vi "TLB Native Dynamic Events ver 0.26d.vi"() -> ()   [LabVIEW 2018] (continued)
                    n435 = for {
                      tunnel: string[] ["START TIMER", "OPEN CLAW", ""] ("element") -> [w1149] mode=indexing
                      shift-right: [w1151] -> w1148
                      shift-left: w1146 -> [w1150]
                      n436 = Enqueue Element(queue=w1150, element=w1149) -> (queue out=w1151:refnum<queue>)  [unwired: 2 in, 2 out]
                    }
                  }
                  frame True {
                    n437 = for {
                      shift-right: [w1156] -> w1154
                      shift-left: w1152 -> [w1157]
                      tunnel: string[] ["CAM CLOSE", "", ""] -> [w1155] mode=indexing
                      n438 = Enqueue Element(queue=w1157, element=w1155) -> (queue out=w1156:refnum<queue>)  [unwired: 2 in, 2 out]
                    }
                  }
                }
                n439 = Or(x=w1135, y=w1140) -> (x .or. y?=w1142:bool)
                n440 = Select(t=State_Type_Definitions,_for_0.26g_versions_and_later_2."True Stop" ("Enum"), s=w1140, f=State_Type_Definitions,_for_0.26g_versions_and_later_2."True Stop" ("Enum")) -> (s? t:f=w1137:T18)
                n441 = Select(t=w1137, s=w1142, f=State_Type_Definitions,_for_0.26g_versions_and_later_2."Task 5D" ("Enum")) -> (s? t:f=w1141:T18)
              }
              frame "Exit" {
                n442 = for {
                  shift-right: [w1164] -> w1161
                  shift-left: w1158 -> [w1165]
                  tunnel: string[] ["STOP", "RESET ENCODERS", "RESET YAW", "ARDUINO MODE 0"] -> [w1163] mode=indexing
                  n443 = Enqueue Element(queue=w1165, element=w1163) -> (queue out=w1164:refnum<queue>)  [unwired: 2 in, 2 out]
                }
              }
            }
          }
          frame 20 {
            # ">>> yStepper command>>>"
            n444 = Dequeue Element(queue=w1179, timeout in ms (-1)=w1180, error in (no error)=w1181) -> (element=w1183:T10)  [unwired: 3 out]
            n445 = formula code="if (pos < 100)\ny = 41;\n\nelse if (pos >= 100 && pos <= 140)\ny = 30;\n\nelse if (pos >= 141 && pos <= 170)\ny = 25;\n\nelse if (pos >= 171 &&pos <= 180) \ny = 20;\n\nelse if (pos >= 181&& pos <= 200)\ny = 15;\n\nelse if (pos >= 201 && pos <= 230)\ny = 10;\n\nelse if (pos >= 231 && pos <= 320)\ny = 8;\n\nelse if (pos > 320)\ny = 0;"("pos"=w1171) -> ("y"=w1174:dbl)
            n446 = To Unsigned Byte Integer(number=w1174) -> (unsigned 8bit integer=w1169:u8)
            n447 = Equal?(x=w1170, y=w1169) -> (x = y?=w1168:bool)
            n448 = case shown="\"Start Task 1\", Default" w1183 {
              tunnel: [w1190 State_Type_Definitions,_for_0.26g_versions_and_later_2."True Stop" ("Enum")] -> w1177
              tunnel: [w1193 w1210] -> w1175
              tunnel: [State_Type_Definitions,_for_0.26g_versions_and_later_2."Idle" ("Enum") State_Type_Definitions,_for_0.26g_versions_and_later_2."Shutdown" ("Enum")] -> w1176
              tunnel: w1182 -> [w1189 _]
              tunnel: w1178 -> [w1185 w1207]
              tunnel: w1168 -> [w1184 _]
              frame "Start Task 1", Default {
                # ">> T: Breaks out of state loop; F: Stays in loop>>"
                # ">> Manual override >>"
                # ">> Checks if time is up>>"
                # "Stays in Task 5D until the object is detected"
                # "T: Go back to idle, F: Continue with task\""
                # ">> Manual override >>"
                n449 = case shown="False" w1184 {
                  tunnel: [w1197 w1203] -> w1193
                  tunnel: w1185 -> [w1195 w1201]
                  frame False {
                    n450 = for {
                      tunnel: string[] ["READ STEPPER VALUES", "Y STEPPER CONTROL", ""] ("element") -> [w1198] mode=indexing
                      shift-right: [w1200] -> w1197
                      shift-left: w1195 -> [w1199]
                      n451 = Enqueue Element(queue=w1199, element=w1198) -> (queue out=w1200:refnum<queue>)  [unwired: 2 in, 2 out]
                    }
                  }
                  frame True {
                    n452 = for {
                      shift-right: [w1205] -> w1203
                      shift-left: w1201 -> [w1206]
                      tunnel: string[] ["CAM CLOSE", "DISPOSE BUFFERS", ""] -> [w1204] mode=indexing
                      n453 = Enqueue Element(queue=w1206, element=w1204) -> (queue out=w1205:refnum<queue>)  [unwired: 2 in, 2 out]
                    }
                  }
                }
                n454 = Or(x=w1184, y=w1189) -> (x .or. y?=w1191:bool)
                n455 = Select(t=State_Type_Definitions,_for_0.26g_versions_and_later_2."True Stop" ("Enum"), s=w1189, f=State_Type_Definitions,_for_0.26g_versions_and_later_2."Task 5F: ARM GRAB HEIGHT" ("Enum")) -> (s? t:f=w1186:T18)
                n456 = Select(t=w1186, s=w1191, f=State_Type_Definitions,_for_0.26g_versions_and_later_2."Task 5E: POSITION ARM" ("Enum")) -> (s? t:f=w1190:T18)
              }
              frame "Exit" {
                n457 = for {
                  shift-right: [w1213] -> w1210
                  shift-left: w1207 -> [w1214]
                  tunnel: string[] ["STOP", "RESET ENCODERS", "RESET YAW", "ARDUINO MODE 0"] -> [w1212] mode=indexing
                  n458 = Enqueue Element(queue=w1214, element=w1212) -> (queue out=w1213:refnum<queue>)  [unwired: 2 in, 2 out]
                }
              }
            }
            n459 = Bundle By Name(cluster=w1173, "yStepper desired"=w1169) -> (w1172:T20)
          }
          frame 21 {
            # ">>> Motor control cluster >>>"
            # ">>> yStepper command>>>"
            # ">> Manual override >>"
            n460 = Dequeue Element(queue=w1225, timeout in ms (-1)=w1224, error in (no error)=w1226) -> (element=w1223:T10)  [unwired: 3 out]
            n461 = Equal?(x=w1222, y=u8 1) -> (x = y?=w1220:bool)
            n462 = case shown="\"Start Task 1\", Default" w1223 {
              tunnel: [w1236 State_Type_Definitions,_for_0.26g_versions_and_later_2."True Stop" ("Enum")] -> w1227
              tunnel: [w1239 w1256] -> w1228
              tunnel: [State_Type_Definitions,_for_0.26g_versions_and_later_2."Idle" ("Enum") State_Type_Definitions,_for_0.26g_versions_and_later_2."Shutdown" ("Enum")] -> w1229
              tunnel: w1220 -> [w1235 _]
              tunnel: w1219 -> [w1234 _]
              tunnel: w1218 -> [w1230 w1253]
              frame "Start Task 1", Default {
                # "Stays in Task 5F until stepper reaches desired \nheight"
                # "T: Go back to idle, F: Continue with task\""
                # ">> Manual override >>"
                n463 = case shown="True" w1235 {
                  tunnel: [w1243 w1249] -> w1239
                  tunnel: w1230 -> [w1241 w1247]
                  frame False {
                    n464 = for {
                      tunnel: string[] ["Z STEPPER GRAB HEIGHT", "READ STEPPER VALUES"] ("element") -> [w1244] mode=indexing
                      shift-right: [w1246] -> w1243
                      shift-left: w1241 -> [w1245]
                      n465 = Enqueue Element(queue=w1245, element=w1244) -> (queue out=w1246:refnum<queue>)  [unwired: 2 in, 2 out]
                    }
                  }
                  frame True {
                    n466 = for {
                      shift-right: [w1251] -> w1249
                      shift-left: w1247 -> [w1252]
                      tunnel: string[] ["SET TIMER 5", "CLOSE CLAW", ""] -> [w1250] mode=indexing
                      n467 = Enqueue Element(queue=w1252, element=w1250) -> (queue out=w1251:refnum<queue>)  [unwired: 2 in, 2 out]
                    }
                  }
                }
                n468 = Or(x=w1235, y=w1234) -> (x .or. y?=w1237:bool)
                n469 = Select(t=State_Type_Definitions,_for_0.26g_versions_and_later_2."True Stop" ("Enum"), s=w1234, f=State_Type_Definitions,_for_0.26g_versions_and_later_2."Task 5G: CLOSE CLAW" ("Enum")) -> (s? t:f=w1231:T18)
                n470 = Select(t=w1231, s=w1237, f=State_Type_Definitions,_for_0.26g_versions_and_later_2."Task 5F: ARM GRAB HEIGHT" ("Enum")) -> (s? t:f=w1236:T18)
              }
              frame "Exit" {
                n471 = for {
                  shift-right: [w1259] -> w1256
                  shift-left: w1253 -> [w1260]
                  tunnel: string[] ["STOP", "RESET ENCODERS", "RESET YAW", "ARDUINO MODE 0"] -> [w1258] mode=indexing
                  n472 = Enqueue Element(queue=w1260, element=w1258) -> (queue out=w1259:refnum<queue>)  [unwired: 2 in, 2 out]
                }
              }
            }
          }
          frame 22 {
            # ">>> yStepper command>>>"
            # ">> Manual override >>"
            n473 = Dequeue Element(queue=w1271, timeout in ms (-1)=w1270, error in (no error)=w1269) -> (element=w1268:T10)  [unwired: 3 out]
            n474 = case shown="\"Start Task 1\", Default" w1268 {
              tunnel: [w1280 State_Type_Definitions,_for_0.26g_versions_and_later_2."True Stop" ("Enum")] -> w1273
              tunnel: [w1283 w1300] -> w1266
              tunnel: [State_Type_Definitions,_for_0.26g_versions_and_later_2."Idle" ("Enum") State_Type_Definitions,_for_0.26g_versions_and_later_2."Shutdown" ("Enum")] -> w1265
              tunnel: w1267 -> [w1274 _]
              tunnel: w1272 -> [w1279 w1297]
              tunnel: w1263 -> [w1278 _]
              frame "Start Task 1", Default {
                # ">> Is time up? >>"
                # "Determines if object is in range to pick up"
                # ">> Manual override >>"
                n475 = case shown="True" w1278 {
                  tunnel: [w1287 w1293] -> w1283
                  tunnel: w1279 -> [w1285 w1291]
                  frame False {
                    n476 = for {
                      tunnel: string[] ["CLOSE CLAW", "START TIMER"] ("element") -> [w1288] mode=indexing
                      shift-right: [w1290] -> w1287
                      shift-left: w1285 -> [w1289]
                      n477 = Enqueue Element(queue=w1289, element=w1288) -> (queue out=w1290:refnum<queue>)  [unwired: 2 in, 2 out]
                    }
                  }
                  frame True {
                    n478 = for {
                      shift-right: [w1295] -> w1293
                      shift-left: w1291 -> [w1296]
                      tunnel: string[] ["READ STEPPER VALUES", "", ""] -> [w1294] mode=indexing
                      n479 = Enqueue Element(queue=w1296, element=w1294) -> (queue out=w1295:refnum<queue>)  [unwired: 2 in, 2 out]
                    }
                  }
                }
                n480 = Or(x=w1278, y=w1274) -> (x .or. y?=w1281:bool)
                n481 = Select(t=State_Type_Definitions,_for_0.26g_versions_and_later_2."True Stop" ("Enum"), s=w1274, f=State_Type_Definitions,_for_0.26g_versions_and_later_2."Task 5H: RAISE ARM" ("Enum")) -> (s? t:f=w1276:T18)
                n482 = Select(t=w1276, s=w1281, f=State_Type_Definitions,_for_0.26g_versions_and_later_2."Task 5G: CLOSE CLAW" ("Enum")) -> (s? t:f=w1280:T18)
              }
              frame "Exit" {
                n483 = for {
                  shift-right: [w1303] -> w1300
                  shift-left: w1297 -> [w1304]
                  tunnel: string[] ["STOP", "RESET ENCODERS", "RESET YAW", "ARDUINO MODE 0"] -> [w1302] mode=indexing
                  n484 = Enqueue Element(queue=w1304, element=w1302) -> (queue out=w1303:refnum<queue>)  [unwired: 2 in, 2 out]
                }
              }
            }
          }
          frame 23 {
            # ">>> yStepper command>>>"
            # ">> Manual override >>"
            n485 = Dequeue Element(queue=w1315, timeout in ms (-1)=w1314, error in (no error)=w1316) -> (element=w1313:T10)  [unwired: 3 out]
            n486 = Equal?(x=w1312, y=u8 60) -> (x = y?=w1310:bool)
            n487 = case shown="\"Start Task 1\", Default" w1313 {
              tunnel: [w1326 State_Type_Definitions,_for_0.26g_versions_and_later_2."True Stop" ("Enum")] -> w1317
              tunnel: [w1329 w1346] -> w1318
              tunnel: [State_Type_Definitions,_for_0.26g_versions_and_later_2."Idle" ("Enum") State_Type_Definitions,_for_0.26g_versions_and_later_2."Shutdown" ("Enum")] -> w1319
              tunnel: w1310 -> [w1325 _]
              tunnel: w1309 -> [w1324 _]
              tunnel: w1308 -> [w1320 w1343]
              frame "Start Task 1", Default {
                # "Stays in Task 5_A until stepper reaches desired \nheight"
                # "T: Go back to idle, F: Continue with task\""
                # ">> Manual override >>"
                n488 = case shown="False" w1325 {
                  tunnel: [w1333 w1339] -> w1329
                  tunnel: w1320 -> [w1331 w1337]
                  frame False {
                    n489 = for {
                      tunnel: string[] ["Z STEPPER CAM HEIGHT", "READ STEPPER VALUES"] ("element") -> [w1334] mode=indexing
                      shift-right: [w1336] -> w1333
                      shift-left: w1331 -> [w1335]
                      n490 = Enqueue Element(queue=w1335, element=w1334) -> (queue out=w1336:refnum<queue>)  [unwired: 2 in, 2 out]
                    }
                  }
                  frame True {
                    n491 = for {
                      shift-right: [w1341] -> w1339
                      shift-left: w1337 -> [w1342]
                      tunnel: string[] ["ARDUINO - ULTRASONIC", "READ ULTRASONIC", ""] -> [w1340] mode=indexing
                      n492 = Enqueue Element(queue=w1342, element=w1340) -> (queue out=w1341:refnum<queue>)  [unwired: 2 in, 2 out]
                    }
                  }
                }
                n493 = Or(x=w1325, y=w1324) -> (x .or. y?=w1327:bool)
                n494 = Select(t=State_Type_Definitions,_for_0.26g_versions_and_later_2."True Stop" ("Enum"), s=w1324, f=State_Type_Definitions,_for_0.26g_versions_and_later_2."True Stop" ("Enum")) -> (s? t:f=w1321:T18)
                n495 = Select(t=w1321, s=w1327, f=State_Type_Definitions,_for_0.26g_versions_and_later_2."Task 5H: RAISE ARM" ("Enum")) -> (s? t:f=w1326:T18)
              }
              frame "Exit" {
                n496 = for {
                  shift-right: [w1349] -> w1346
                  shift-left: w1343 -> [w1350]
                  tunnel: string[] ["STOP", "RESET ENCODERS", "RESET YAW", "ARDUINO MODE 0"] -> [w1348] mode=indexing
                  n497 = Enqueue Element(queue=w1350, element=w1348) -> (queue out=w1349:refnum<queue>)  [unwired: 2 in, 2 out]
                }
              }
            }
          }
          frame 24 {
            # ">>> yStepper command>>>"
            n498 = Dequeue Element(queue=w1360, timeout in ms (-1)=w1359, error in (no error)=w1358) -> (element=w1365:T10)  [unwired: 3 out]
            n499 = Equal?(x=w1356, y=u8 60) -> (x = y?=w1355:bool)
            n500 = case shown="\"Start Task 1\", Default" w1365 {
              tunnel: [w1372 State_Type_Definitions,_for_0.26g_versions_and_later_2."True Stop" ("Enum")] -> w1363
              tunnel: [w1371 w1389] -> w1362
              tunnel: [State_Type_Definitions,_for_0.26g_versions_and_later_2."Idle" ("Enum") State_Type_Definitions,_for_0.26g_versions_and_later_2."Shutdown" ("Enum")] -> w1364
              tunnel: w1361 -> [w1367 _]
              tunnel: w1357 -> [w1369 _]
              tunnel: w1355 -> [w1366 _]
              frame "Start Task 1", Default {
                n501 = case shown="False" w1366 {
                  tunnel: [w1377 w1383] -> w1371
                  tunnel: w1369 -> [w1375 w1381]
                  frame False {
                    n502 = for {
                      tunnel: string[] ["Z STEPPER CAM HEIGHT", "READ STEPPER VALUES"] ("element") -> [w1378] mode=indexing
                      shift-right: [w1380] -> w1377
                      shift-left: w1375 -> [w1379]
                      n503 = Enqueue Element(queue=w1379, element=w1378) -> (queue out=w1380:refnum<queue>)  [unwired: 2 in, 2 out]
                    }
                  }
                  frame True {
                    n504 = for {
                      shift-right: [w1385] -> w1383
                      shift-left: w1381 -> [w1386]
                      tunnel: string[] ["CAM ACQ", "OPEN LOG CAM"] -> [w1384] mode=indexing
                      n505 = Enqueue Element(queue=w1386, element=w1384) -> (queue out=w1385:refnum<queue>)  [unwired: 2 in, 2 out]
                    }
                  }
                }
                n506 = Or(x=w1366, y=w1367) -> (x .or. y?=w1368:bool)
                n507 = Select(t=State_Type_Definitions,_for_0.26g_versions_and_later_2."Task 6_B" ("Enum"), s=w1368, f=State_Type_Definitions,_for_0.26g_versions_and_later_2."Task 6_A" ("Enum")) -> (s? t:f=w1372:T18)
              }
              frame "Exit" {
                n508 = for {
                  shift-right: [w1392] -> w1389
                  shift-left: _ -> [w1393]
                  tunnel: string[] ["STOP", "RESET ENCODERS", "RESET YAW", "ARDUINO MODE 0"] -> [w1391] mode=indexing
                  n509 = Enqueue Element(queue=w1393, element=w1391) -> (queue out=w1392:refnum<queue>)  [unwired: 2 in, 2 out]
                }
              }
            }
          }
          frame 25 {
            # ">>> yStepper command>>>"
            n510 = Dequeue Element(queue=w1405, timeout in ms (-1)=w1403, error in (no error)=w1404) -> (element=w1402:T10)  [unwired: 3 out]
            n511 = case shown="\"Start Task 1\", Default" w1402 {
              tunnel: [w1412 State_Type_Definitions,_for_0.26g_versions_and_later_2."True Stop" ("Enum")] -> w1398
              tunnel: [w1411 w1430] -> w1406
              tunnel: [State_Type_Definitions,_for_0.26g_versions_and_later_2."Idle" ("Enum") State_Type_Definitions,_for_0.26g_versions_and_later_2."Shutdown" ("Enum")] -> w1399
              tunnel: w1401 -> [w1407 _]
              tunnel: w1400 -> [w1409 _]
              tunnel: w1397 -> [w1408 w1427]
              frame "Start Task 1", Default {
                # ">> Manual override >>"
                n512 = case shown="False" w1409 {
                  tunnel: [w1417 w1423] -> w1411
                  tunnel: w1408 -> [w1416 w1421]
                  frame False {
                    n513 = for {
                      shift-right: [w1420] -> w1417
                      shift-left: w1416 -> [w1419]
                      tunnel: string[] ["CAM ACQ", "PROCESS IMAGE", "OPEN CLAW"] -> [w1418] mode=indexing
                      n514 = Enqueue Element(queue=w1419, element=w1418) -> (queue out=w1420:refnum<queue>)  [unwired: 2 in, 2 out]
                    }
                  }
                  frame True {
                    n515 = for {
                      shift-right: [w1425] -> w1423
                      shift-left: w1421 -> [w1426]
                      tunnel: string[] ["CAM ACQ", "PROCESS IMAGE", "CLOSE CLAW"] -> [w1424] mode=indexing
                      n516 = Enqueue Element(queue=w1426, element=w1424) -> (queue out=w1425:refnum<queue>)  [unwired: 2 in, 2 out]
                    }
                  }
                }
                n517 = Select(t=State_Type_Definitions,_for_0.26g_versions_and_later_2."True Stop" ("Enum"), s=w1407, f=State_Type_Definitions,_for_0.26g_versions_and_later_2."Task 6_B" ("Enum")) -> (s? t:f=w1412:T18)
              }
              frame "Exit" {
                # ">> State after true stop >>"
                # ">> Goes to true stop >>"
                n518 = for {
                  shift-right: [w1433] -> w1430
                  shift-left: w1427 -> [w1434]
                  tunnel: string[] ["STOP", "RESET ENCODERS", "RESET YAW", ""] -> [w1432] mode=indexing
                  n519 = Enqueue Element(queue=w1434, element=w1432) -> (queue out=w1433:refnum<queue>)  [unwired: 2 in, 2 out]
                }
              }
            }
          }
          frame 26 {
          }
          frame 27 {
            # ">>> Motor control cluster >>>"
            # ">>> yStepper command>>>"
            # ">> Manual override >>"
            n520 = Dequeue Element(queue=w1451, timeout in ms (-1)=w1450, error in (no error)=w1452) -> (element=w1449:T10)  [unwired: 3 out]
            n521 = Equal?(x=w1448, y=u8 60) -> (x = y?=w1446:bool)
            n522 = case shown="\"Start Task 1\", Default" w1449 {
              tunnel: [w1462 State_Type_Definitions,_for_0.26g_versions_and_later_2."True Stop" ("Enum")] -> w1453
              tunnel: [w1465 w1482] -> w1454
              tunnel: [State_Type_Definitions,_for_0.26g_versions_and_later_2."Idle" ("Enum") State_Type_Definitions,_for_0.26g_versions_and_later_2."Shutdown" ("Enum")] -> w1455
              tunnel: w1446 -> [w1461 _]
              tunnel: w1445 -> [w1460 _]
              tunnel: w1444 -> [w1456 w1479]
              frame "Start Task 1", Default {
                # "Stays in Task 5_A until stepper reaches desired \nheight"
                # "T: Go back to idle, F: Continue with task\""
                # ">> Manual override >>"
                n523 = case shown="False" w1461 {
                  tunnel: [w1469 w1475] -> w1465
                  tunnel: w1456 -> [w1467 w1473]
                  frame False {
                    n524 = for {
                      tunnel: string[] ["Z STEPPER CAM HEIGHT", "READ STEPPER VALUES"] ("element") -> [w1470] mode=indexing
                      shift-right: [w1472] -> w1469
                      shift-left: w1467 -> [w1471]
                      n525 = Enqueue Element(queue=w1471, element=w1470) -> (queue out=w1472:refnum<queue>)  [unwired: 2 in, 2 out]
                    }
                  }
                  frame True {
                    n526 = for {
                      shift-right: [w1477] -> w1475
                      shift-left: w1473 -> [w1478]
                      tunnel: string[] ["ARDUINO - ULTRASONIC", "READ ULTRASONIC", ""] -> [w1476] mode=indexing
                      n527 = Enqueue Element(queue=w1478, element=w1476) -> (queue out=w1477:refnum<queue>)  [unwired: 2 in, 2 out]
                    }
                  }
                }
                n528 = Or(x=w1461, y=w1460) -> (x .or. y?=w1463:bool)
                n529 = Select(t=State_Type_Definitions,_for_0.26g_versions_and_later_2."True Stop" ("Enum"), s=w1460, f=State_Type_Definitions,_for_0.26g_versions_and_later_2."Task 8B: MOVE TO BOX" ("Enum")) -> (s? t:f=w1457:T18)
                n530 = Select(t=w1457, s=w1463, f=State_Type_Definitions,_for_0.26g_versions_and_later_2."Task 8A: RAISE ARM" ("Enum")) -> (s? t:f=w1462:T18)
              }
              frame "Exit" {
                n531 = for {
                  shift-right: [w1485] -> w1482
                  shift-left: w1479 -> [w1486]
                  tunnel: string[] ["STOP", "RESET ENCODERS", "RESET YAW", "ARDUINO MODE 0"] -> [w1484] mode=indexing
                  n532 = Enqueue Element(queue=w1486, element=w1484) -> (queue out=w1485:refnum<queue>)  [unwired: 2 in, 2 out]
                }
              }
            }
          }
          frame 28 {
            w1494 = u8 15 ("y")
            # ">>> yStepper command>>>"
            n533 = Less?(x=w1491, y=w1494) -> (x < y?=w1492:bool)
            n534 = Dequeue Element(queue=w1498, timeout in ms (-1)=w1497, error in (no error)=w1499) -> (element=w1496:T10)  [unwired: 3 out]
            n535 = Less?(x=w1490, y=w1494) -> (x < y?=w1493:bool)
            n536 = And(x=w1493, y=w1492) -> (x .and. y?=w1489:bool)
            n537 = case shown="\"Start Task 1\", Default" w1496 {
              tunnel: [w1511 State_Type_Definitions,_for_0.26g_versions_and_later_2."True Stop" ("Enum")] -> w1501
              tunnel: [w1514 w1531] -> w1500
              tunnel: [State_Type_Definitions,_for_0.26g_versions_and_later_2."Idle" ("Enum") State_Type_Definitions,_for_0.26g_versions_and_later_2."Shutdown" ("Enum")] -> w1502
              tunnel: w1504 -> [w1510 _]
              tunnel: w1503 -> [w1506 w1528]
              tunnel: w1489 -> [w1505 _]
              frame "Start Task 1", Default {
                # "Stays in Task 5_B to capture image over 5 seconds"
                # "T: Go back to idle, F: Continue with task\""
                # ">> Manual override >>"
                n538 = case shown="True" w1505 {
                  tunnel: [w1518 w1524] -> w1514
                  tunnel: w1506 -> [w1516 w1522]
                  frame False {
                    n539 = for {
                      tunnel: string[] ["FORWARD", "READ ULTRASONIC", "READ NAVX"] ("element") -> [w1519] mode=indexing
                      shift-right: [w1521] -> w1518
                      shift-left: w1516 -> [w1520]
                      n540 = Enqueue Element(queue=w1520, element=w1519) -> (queue out=w1521:refnum<queue>)  [unwired: 2 in, 2 out]
                    }
                  }
                  frame True {
                    n541 = for {
                      shift-right: [w1526] -> w1524
                      shift-left: w1522 -> [w1527]
                      tunnel: string[] ["STOP", "RESET ENCODERS", "OPEN LOG CAM", "SET TIMER 2", "OPEN IMAQ REF"] -> [w1525] mode=indexing
                      n542 = Enqueue Element(queue=w1527, element=w1525) -> (queue out=w1526:refnum<queue>)  [unwired: 2 in, 2 out]
                    }
                  }
                }
                n543 = Or(x=w1505, y=w1510) -> (x .or. y?=w1512:bool)
                n544 = Select(t=State_Type_Definitions,_for_0.26g_versions_and_later_2."True Stop" ("Enum"), s=w1510, f=State_Type_Definitions,_for_0.26g_versions_and_later_2."Task 8C: CAM BURST" ("Enum")) -> (s? t:f=w1507:T18)
                n545 = Select(t=w1507, s=w1512, f=State_Type_Definitions,_for_0.26g_versions_and_later_2."Task 8B: MOVE TO BOX" ("Enum")) -> (s? t:f=w1511:T18)
              }
              frame "Exit" {
                n546 = for {
                  shift-right: [w1534] -> w1531
                  shift-left: w1528 -> [w1535]
                  tunnel: string[] ["STOP", "RESET ENCODERS", "RESET YAW", "ARDUINO MODE 0"] -> [w1533] mode=indexing
                  n547 = Enqueue Element(queue=w1535, element=w1533) -> (queue out=w1534:refnum<queue>)  [unwired: 2 in, 2 out]
                }
              }
            }
          }
          frame 29 {
            # ">>> Motor control cluster >>>"
            # ">>> yStepper command>>>"
            # ">> Manual override >>"
            n548 = Dequeue Element(queue=w1546, timeout in ms (-1)=w1545, error in (no error)=w1544) -> (element=w1543:T10)  [unwired: 3 out]
            n549 = case shown="\"Start Task 1\", Default" w1543 {
              tunnel: [w1555 State_Type_Definitions,_for_0.26g_versions_and_later_2."True Stop" ("Enum")] -> w1548
              tunnel: [w1558 w1575] -> w1541
              tunnel: [State_Type_Definitions,_for_0.26g_versions_and_later_2."Idle" ("Enum") State_Type_Definitions,_for_0.26g_versions_and_later_2."Shutdown" ("Enum")] -> w1540
              tunnel: w1542 -> [w1549 _]
              tunnel: w1547 -> [w1554 w1572]
              tunnel: w1538 -> [w1553 _]
              frame "Start Task 1", Default {
                # ">> Is time up? >>"
                # "Determines if object is in range to pick up"
                # ">> Manual override >>"
                n550 = case shown="True" w1553 {
                  tunnel: [w1562 w1568] -> w1558
                  tunnel: w1554 -> [w1560 w1566]
                  frame False {
                    n551 = for {
                      tunnel: string[] ["CAM ACQ", "START TIMER"] ("element") -> [w1563] mode=indexing
                      shift-right: [w1565] -> w1562
                      shift-left: w1560 -> [w1564]
                      n552 = Enqueue Element(queue=w1564, element=w1563) -> (queue out=w1565:refnum<queue>)  [unwired: 2 in, 2 out]
                    }
                  }
                  frame True {
                    n553 = for {
                      shift-right: [w1570] -> w1568
                      shift-left: w1566 -> [w1571]
                      tunnel: string[] ["CAM CLOSE", "PROCESS IMAGE", "SET TIMER 5"] -> [w1569] mode=indexing
                      n554 = Enqueue Element(queue=w1571, element=w1569) -> (queue out=w1570:refnum<queue>)  [unwired: 2 in, 2 out]
                    }
                  }
                }
                n555 = Or(x=w1553, y=w1549) -> (x .or. y?=w1556:bool)
                n556 = Select(t=State_Type_Definitions,_for_0.26g_versions_and_later_2."True Stop" ("Enum"), s=w1549, f=State_Type_Definitions,_for_0.26g_versions_and_later_2."Task 8D: PROCESS IMAGE" ("Enum")) -> (s? t:f=w1551:T18)
                n557 = Select(t=w1551, s=w1556, f=State_Type_Definitions,_for_0.26g_versions_and_later_2."Task 8C: CAM BURST" ("Enum")) -> (s? t:f=w1555:T18)
              }
              frame "Exit" {
                n558 = for {
                  shift-right: [w1578] -> w1575
                  shift-left: w1572 -> [w1579]
                  tunnel: string[] ["STOP", "RESET ENCODERS", "RESET YAW", "ARDUINO MODE 0"] -> [w1577] mode=indexing
                  n559 = Enqueue Element(queue=w1579, element=w1577) -> (queue out=w1578:refnum<queue>)  [unwired: 2 in, 2 out]
                }
              }
            }
          }
          frame 30 {
            # ">>> yStepper command>>>"
            n560 = Dequeue Element(queue=w1587, timeout in ms (-1)=w1586, error in (no error)=w1585) -> (element=w1584:T10)  [unwired: 3 out]
            n561 = case shown="\"Start Task 1\", Default" w1584 {
              tunnel: [w1599 State_Type_Definitions,_for_0.26g_versions_and_later_2."True Stop" ("Enum")] -> w1591
              tunnel: [w1602 w1619] -> w1590
              tunnel: [State_Type_Definitions,_for_0.26g_versions_and_later_2."Idle" ("Enum") State_Type_Definitions,_for_0.26g_versions_and_later_2."Shutdown" ("Enum")] -> w1592
              tunnel: w1588 -> [w1598 _]
              tunnel: w1589 -> [w1594 w1616]
              tunnel: w1582 -> [w1593 _]
              frame "Start Task 1", Default {
                # ">> T: Breaks out of state loop; F: Stays in loop>>"
                # ">> Manual override >>"
                # ">> Checks if time is up>>"
                # "Stays in Task 5D until the object is detected"
                # "T: Go back to idle, F: Continue with task\""
                # ">> Manual override >>"
                n562 = case shown="False" w1593 {
                  tunnel: [w1606 w1612] -> w1602
                  tunnel: w1594 -> [w1604 w1610]
                  frame False {
                    n563 = for {
                      tunnel: string[] ["START TIMER", "PROCESS IMAGE", ""] ("element") -> [w1607] mode=indexing
                      shift-right: [w1609] -> w1606
                      shift-left: w1604 -> [w1608]
                      n564 = Enqueue Element(queue=w1608, element=w1607) -> (queue out=w1609:refnum<queue>)  [unwired: 2 in, 2 out]
                    }
                  }
                  frame True {
                    n565 = for {
                      shift-right: [w1614] -> w1612
                      shift-left: w1610 -> [w1615]
                      tunnel: string[] ["RESET ENCODERS", "", ""] -> [w1613] mode=indexing
                      n566 = Enqueue Element(queue=w1615, element=w1613) -> (queue out=w1614:refnum<queue>)  [unwired: 2 in, 2 out]
                    }
                  }
                }
                n567 = Or(x=w1593, y=w1598) -> (x .or. y?=w1600:bool)
                n568 = Select(t=State_Type_Definitions,_for_0.26g_versions_and_later_2."True Stop" ("Enum"), s=w1598, f=State_Type_Definitions,_for_0.26g_versions_and_later_2."Task 8E: ROBOT ADJUST" ("Enum")) -> (s? t:f=w1595:T18)
                n569 = Select(t=w1595, s=w1600, f=State_Type_Definitions,_for_0.26g_versions_and_later_2."Task 8D: PROCESS IMAGE" ("Enum")) -> (s? t:f=w1599:T18)
              }
              frame "Exit" {
                n570 = for {
                  shift-right: [w1622] -> w1619
                  shift-left: w1616 -> [w1623]
                  tunnel: string[] ["STOP", "RESET ENCODERS", "RESET YAW", "ARDUINO MODE 0"] -> [w1621] mode=indexing
                  n571 = Enqueue Element(queue=w1623, element=w1621) -> (queue out=w1622:refnum<queue>)  [unwired: 2 in, 2 out]
                }
              }
            }
          }
          frame 31 {
            # ">>> Motor control cluster >>>"
            # ">>> yStepper command>>>"
            n572 = Dequeue Element(queue=w1640, timeout in ms (-1)=w1639, error in (no error)=w1638) -> (element=w1637:T10)  [unwired: 3 out]
            n573 = Subtract(x=w1635, y=300.0) -> (x-y=w1633:dbl)
            n574 = formula code="if (error <= -61&&error > -300){\ndistance = -15;\nxSpeed = -30;\n}\n\nelse if (error <= -51 && error >= -60){\ndistance = -10;\nxSpeed = -30;\n}\n\nelse if (error >= -50 && error <= 50){\ndistance = 0;\nxSpeed = 0;\n}\n\nelse if (error >= 51 && error <= 80){\ndistance = 10;\nxSpeed = 30;\n}\n\nelse if (error >= 81 && error <= 100){\ndistance = 15;\nxSpeed = 30;\n}\n\nelse if (error >= 101 && error <= 120){\ndistance = 20;\nxSpeed = 30;\n}\n\nelse if (error >= 121 && error < 300){\ndistance = 25;\nxSpeed = 30;\n}\n\nelse{\ndistance = 0;\nxSpeed = 0;\n}"("error"=w1633) -> ("distance"=w1628:dbl, "xSpeed"=w1630:dbl)
            n575 = formula code="if (target > 0){\nif (current  >= target)\noutput = 1;\n\nelse if (current != target)\noutput = 0;\n}\n\nelse if (target == 0){\nif (current == target)\noutput = 1;\n\nelse if (current != target)\noutput = 0;\n}\n\nelse if (target < 0){\nif (current <= target)\noutput = 1;\n\nelse if (current != target)\noutput = 0;\n}\n\nelse if (current != target)\noutput = 0;"("target"=w1628, "current"=w1629) -> ("output"=w1627:dbl)
            n576 = Bundle By Name(cluster=w1632, "xSpeed"=w1630) -> (w1631:T19)
            n577 = Equal?(x=w1627, y=1.0) -> (x = y?=w1625:bool)
            n578 = case shown="\"Start Task 1\", Default" w1637 {
              tunnel: [w1652 State_Type_Definitions,_for_0.26g_versions_and_later_2."True Stop" ("Enum")] -> w1644
              tunnel: [w1655 w1672] -> w1643
              tunnel: [State_Type_Definitions,_for_0.26g_versions_and_later_2."Idle" ("Enum") State_Type_Definitions,_for_0.26g_versions_and_later_2."Shutdown" ("Enum")] -> w1645
              tunnel: w1641 -> [w1651 _]
              tunnel: w1642 -> [w1647 w1669]
              tunnel: w1625 -> [w1646 _]
              frame "Start Task 1", Default {
                # ">> T: Breaks out of state loop; F: Stays in loop>>"
                # ">> Manual override >>"
                # ">> Checks if time is up>>"
                # "Stays in Task 5D until the object is detected"
                # "T: Go back to idle, F: Continue with task\""
                # ">> Manual override >>"
                n579 = case shown="True" w1646 {
                  tunnel: [w1659 w1665] -> w1655
                  tunnel: w1647 -> [w1657 w1663]
                  frame False {
                    n580 = for {
                      tunnel: string[] ["X AXIS - SLOW", "READ ENCODERS", "READ NAVX"] ("element") -> [w1660] mode=indexing
                      shift-right: [w1662] -> w1659
                      shift-left: w1657 -> [w1661]
                      n581 = Enqueue Element(queue=w1661, element=w1660) -> (queue out=w1662:refnum<queue>)  [unwired: 2 in, 2 out]
                    }
                  }
                  frame True {
                    n582 = for {
                      shift-right: [w1667] -> w1665
                      shift-left: w1663 -> [w1668]
                      tunnel: string[] ["SET TIMER 2", "STOP", "READ STEPPER VALUES", ""] -> [w1666] mode=indexing
                      n583 = Enqueue Element(queue=w1668, element=w1666) -> (queue out=w1667:refnum<queue>)  [unwired: 2 in, 2 out]
                    }
                  }
                }
                n584 = Or(x=w1646, y=w1651) -> (x .or. y?=w1653:bool)
                n585 = Select(t=State_Type_Definitions,_for_0.26g_versions_and_later_2."True Stop" ("Enum"), s=w1651, f=State_Type_Definitions,_for_0.26g_versions_and_later_2."Task 8H: ARM ADJUST" ("Enum")) -> (s? t:f=w1648:T18)
                n586 = Select(t=w1648, s=w1653, f=State_Type_Definitions,_for_0.26g_versions_and_later_2."Task 8E: ROBOT ADJUST" ("Enum")) -> (s? t:f=w1652:T18)
              }
              frame "Exit" {
                n587 = for {
                  shift-right: [w1675] -> w1672
                  shift-left: w1669 -> [w1676]
                  tunnel: string[] ["STOP", "RESET ENCODERS", "RESET YAW", "ARDUINO MODE 0"] -> [w1674] mode=indexing
                  n588 = Enqueue Element(queue=w1676, element=w1674) -> (queue out=w1675:refnum<queue>)  [unwired: 2 in, 2 out]
                }
              }
            }
          }
          frame 32 {
            # ">>> Motor control cluster >>>"
            # ">>> yStepper command>>>"
            # ">> Manual override >>"
            n589 = Dequeue Element(queue=w1687, timeout in ms (-1)=w1686, error in (no error)=w1685) -> (element=w1684:T10)  [unwired: 3 out]
            n590 = case shown="\"Start Task 1\", Default" w1684 {
              tunnel: [w1696 State_Type_Definitions,_for_0.26g_versions_and_later_2."True Stop" ("Enum")] -> w1689
              tunnel: [w1699 w1716] -> w1682
              tunnel: [State_Type_Definitions,_for_0.26g_versions_and_later_2."Idle" ("Enum") State_Type_Definitions,_for_0.26g_versions_and_later_2."Shutdown" ("Enum")] -> w1681
              tunnel: w1683 -> [w1690 _]
              tunnel: w1688 -> [w1695 w1713]
              tunnel: w1679 -> [w1694 _]
              frame "Start Task 1", Default {
                # ">> Is time up? >>"
                # "Determines if object is in range to pick up"
                # ">> Manual override >>"
                n591 = case shown="False" w1694 {
                  tunnel: [w1703 w1709] -> w1699
                  tunnel: w1695 -> [w1701 w1707]
                  frame False {
                    n592 = for {
                      tunnel: string[] ["CAM ACQ", "START TIMER"] ("element") -> [w1704] mode=indexing
                      shift-right: [w1706] -> w1703
                      shift-left: w1701 -> [w1705]
                      n593 = Enqueue Element(queue=w1705, element=w1704) -> (queue out=w1706:refnum<queue>)  [unwired: 2 in, 2 out]
                    }
                  }
                  frame True {
                    n594 = for {
                      shift-right: [w1711] -> w1709
                      shift-left: w1707 -> [w1712]
                      tunnel: string[] ["CAM CLOSE", "PROCESS IMAGE", "SET TIMER 3"] -> [w1710] mode=indexing
                      n595 = Enqueue Element(queue=w1712, element=w1710) -> (queue out=w1711:refnum<queue>)  [unwired: 2 in, 2 out]
                    }
                  }
                }
                n596 = Or(x=w1694, y=w1690) -> (x .or. y?=w1697:bool)
                n597 = Select(t=State_Type_Definitions,_for_0.26g_versions_and_later_2."True Stop" ("Enum"), s=w1690, f=State_Type_Definitions,_for_0.26g_versions_and_later_2."Task 8G: PROCESS IMAGE 2" ("Enum")) -> (s? t:f=w1692:T18)
                n598 = Select(t=w1692, s=w1697, f=State_Type_Definitions,_for_0.26g_versions_and_later_2."Task 8F: CAM BURST 2" ("Enum")) -> (s? t:f=w1696:T18)
              }
              frame "Exit" {
                n599 = for {
                  shift-right: [w1719] -> w1716
                  shift-left: w1713 -> [w1720]
                  tunnel: string[] ["STOP", "RESET ENCODERS", "RESET YAW", "ARDUINO MODE 0"] -> [w1718] mode=indexing
                  n600 = Enqueue Element(queue=w1720, element=w1718) -> (queue out=w1719:refnum<queue>)  [unwired: 2 in, 2 out]
                }
              }
            }
          }
          frame 33 {
            # ">>> yStepper command>>>"
            n601 = Dequeue Element(queue=w1728, timeout in ms (-1)=w1727, error in (no error)=w1726) -> (element=w1725:T10)  [unwired: 3 out]
            n602 = case shown="\"Start Task 1\", Default" w1725 {
              tunnel: [w1740 State_Type_Definitions,_for_0.26g_versions_and_later_2."True Stop" ("Enum")] -> w1732
              tunnel: [w1743 w1760] -> w1731
              tunnel: [State_Type_Definitions,_for_0.26g_versions_and_later_2."Idle" ("Enum") State_Type_Definitions,_for_0.26g_versions_and_later_2."Shutdown" ("Enum")] -> w1733
              tunnel: w1729 -> [w1739 _]
              tunnel: w1730 -> [w1735 w1757]
              tunnel: w1723 -> [w1734 _]
              frame "Start Task 1", Default {
                # ">> T: Breaks out of state loop; F: Stays in loop>>"
                # ">> Manual override >>"
                # ">> Checks if time is up>>"
                # "Stays in Task 5D until the object is detected"
                # "T: Go back to idle, F: Continue with task\""
                # ">> Manual override >>"
                n603 = case shown="False" w1734 {
                  tunnel: [w1747 w1753] -> w1743
                  tunnel: w1735 -> [w1745 w1751]
                  frame False {
                    n604 = for {
                      tunnel: string[] ["START TIMER", "PROCESS IMAGE", ""] ("element") -> [w1748] mode=indexing
                      shift-right: [w1750] -> w1747
                      shift-left: w1745 -> [w1749]
                      n605 = Enqueue Element(queue=w1749, element=w1748) -> (queue out=w1750:refnum<queue>)  [unwired: 2 in, 2 out]
                    }
                  }
                  frame True {
                    n606 = for {
                      shift-right: [w1755] -> w1753
                      shift-left: w1751 -> [w1756]
                      tunnel: string[] ["READ STEPPER VALUES", "Y STEPPER CONTROL", ""] -> [w1754] mode=indexing
                      n607 = Enqueue Element(queue=w1756, element=w1754) -> (queue out=w1755:refnum<queue>)  [unwired: 2 in, 2 out]
                    }
                  }
                }
                n608 = Or(x=w1734, y=w1739) -> (x .or. y?=w1741:bool)
                n609 = Select(t=State_Type_Definitions,_for_0.26g_versions_and_later_2."True Stop" ("Enum"), s=w1739, f=State_Type_Definitions,_for_0.26g_versions_and_later_2."Task 8H: ARM ADJUST" ("Enum")) -> (s? t:f=w1736:T18)
                n610 = Select(t=w1736, s=w1741, f=State_Type_Definitions,_for_0.26g_versions_and_later_2."Task 8G: PROCESS IMAGE 2" ("Enum")) -> (s? t:f=w1740:T18)
              }
              frame "Exit" {
                n611 = for {
                  shift-right: [w1763] -> w1760
                  shift-left: w1757 -> [w1764]
                  tunnel: string[] ["STOP", "RESET ENCODERS", "RESET YAW", "ARDUINO MODE 0"] -> [w1762] mode=indexing
                  n612 = Enqueue Element(queue=w1764, element=w1762) -> (queue out=w1763:refnum<queue>)  [unwired: 2 in, 2 out]
                }
              }
            }
          }
          frame 34 {
            # ">>> yStepper command>>>"
            n613 = Dequeue Element(queue=w1778, timeout in ms (-1)=w1779, error in (no error)=w1780) -> (element=w1782:T10)  [unwired: 3 out]
            n614 = formula code="if (pos < 70)\ny = 43;\n\nelse if (pos >= 71 &&pos <= 80)\ny = 40;\n\nelse if (pos >= 81 && pos <= 90)\ny = 38;\n\nelse if (pos >= 91 &&pos <= 120)\ny = 35;\n\nelse if (pos >= 121 && pos <= 140)\ny = 30;\n\nelse if (pos >= 141 && pos <= 170)\ny = 26;\n\nelse if (pos >= 171 &&pos <= 220) \ny = 20;\n\nelse if (pos >= 221&& pos <= 240)\ny = 15;\n\nelse if (pos >= 241 && pos <= 250)\ny = 10;\n\nelse if (pos >= 251)\ny = 0;"("pos"=w1770) -> ("y"=w1773:dbl)
            n615 = To Unsigned Byte Integer(number=w1773) -> (unsigned 8bit integer=w1768:u8)
            n616 = Equal?(x=w1769, y=w1768) -> (x = y?=w1767:bool)
            n617 = case shown="\"Start Task 1\", Default" w1782 {
              tunnel: [w1789 State_Type_Definitions,_for_0.26g_versions_and_later_2."True Stop" ("Enum")] -> w1776
              tunnel: [w1792 w1809] -> w1774
              tunnel: [State_Type_Definitions,_for_0.26g_versions_and_later_2."Idle" ("Enum") State_Type_Definitions,_for_0.26g_versions_and_later_2."Shutdown" ("Enum")] -> w1775
              tunnel: w1781 -> [w1788 _]
              tunnel: w1777 -> [w1784 w1806]
              tunnel: w1767 -> [w1783 _]
              frame "Start Task 1", Default {
                # ">> T: Breaks out of state loop; F: Stays in loop>>"
                # ">> Manual override >>"
                # ">> Checks if time is up>>"
                # "Stays in Task 5D until the object is detected"
                # "T: Go back to idle, F: Continue with task\""
                # ">> Manual override >>"
                n618 = case shown="False" w1783 {
                  tunnel: [w1796 w1802] -> w1792
                  tunnel: w1784 -> [w1794 w1800]
                  frame False {
                    n619 = for {
                      tunnel: string[] ["READ STEPPER VALUES", "Y STEPPER CONTROL", ""] ("element") -> [w1797] mode=indexing
                      shift-right: [w1799] -> w1796
                      shift-left: w1794 -> [w1798]
                      n620 = Enqueue Element(queue=w1798, element=w1797) -> (queue out=w1799:refnum<queue>)  [unwired: 2 in, 2 out]
                    }
                  }
                  frame True {
                    n621 = for {
                      shift-right: [w1804] -> w1802
                      shift-left: w1800 -> [w1805]
                      tunnel: string[] ["DISPOSE BUFFERS", "READ STEPPER VALUES", ""] -> [w1803] mode=indexing
                      n622 = Enqueue Element(queue=w1805, element=w1803) -> (queue out=w1804:refnum<queue>)  [unwired: 2 in, 2 out]
                    }
                  }
                }
                n623 = Or(x=w1783, y=w1788) -> (x .or. y?=w1790:bool)
                n624 = Select(t=State_Type_Definitions,_for_0.26g_versions_and_later_2."True Stop" ("Enum"), s=w1788, f=State_Type_Definitions,_for_0.26g_versions_and_later_2."Task 8I: ARM GRAB HEIGHT" ("Enum")) -> (s? t:f=w1785:T18)
                n625 = Select(t=w1785, s=w1790, f=State_Type_Definitions,_for_0.26g_versions_and_later_2."Task 8H: ARM ADJUST" ("Enum")) -> (s? t:f=w1789:T18)
              }
              frame "Exit" {
                n626 = for {
                  shift-right: [w1812] -> w1809
                  shift-left: w1806 -> [w1813]
                  tunnel: string[] ["STOP", "RESET ENCODERS", "RESET YAW", "ARDUINO MODE 0"] -> [w1811] mode=indexing
                  n627 = Enqueue Element(queue=w1813, element=w1811) -> (queue out=w1812:refnum<queue>)  [unwired: 2 in, 2 out]
                }
              }
            }
            n628 = Bundle By Name(cluster=w1772, "yStepper desired"=w1768) -> (w1771:T20)
          }
          frame 35 {
            # ">>> Motor control cluster >>>"
            # ">>> yStepper command>>>"
            # ">> Manual override >>"
            n629 = Dequeue Element(queue=w1824, timeout in ms (-1)=w1823, error in (no error)=w1825) -> (element=w1822:T10)  [unwired: 3 out]
            n630 = Equal?(x=w1821, y=u8 1) -> (x = y?=w1819:bool)
            n631 = case shown="\"Start Task 1\", Default" w1822 {
              tunnel: [w1835 State_Type_Definitions,_for_0.26g_versions_and_later_2."True Stop" ("Enum")] -> w1826
              tunnel: [w1838 w1855] -> w1827
              tunnel: [State_Type_Definitions,_for_0.26g_versions_and_later_2."Idle" ("Enum") State_Type_Definitions,_for_0.26g_versions_and_later_2."Shutdown" ("Enum")] -> w1828
              tunnel: w1819 -> [w1834 _]
              tunnel: w1818 -> [w1833 _]
              tunnel: w1817 -> [w1829 w1852]
              frame "Start Task 1", Default {
                # "Stays in Task 5F until stepper reaches desired \nheight"
                # "T: Go back to idle, F: Continue with task\""
                # ">> Manual override >>"
                n632 = case shown="True" w1834 {
                  tunnel: [w1842 w1848] -> w1838
                  tunnel: w1829 -> [w1840 w1846]
                  frame False {
                    n633 = for {
                      tunnel: string[] ["Z STEPPER GRAB HEIGHT", "READ STEPPER VALUES"] ("element") -> [w1843] mode=indexing
                      shift-right: [w1845] -> w1842
                      shift-left: w1840 -> [w1844]
                      n634 = Enqueue Element(queue=w1844, element=w1843) -> (queue out=w1845:refnum<queue>)  [unwired: 2 in, 2 out]
                    }
                  }
                  frame True {
                    n635 = for {
                      shift-right: [w1850] -> w1848
                      shift-left: w1846 -> [w1851]
                      tunnel: string[] ["SET TIMER 2", "CLOSE CLAW", ""] -> [w1849] mode=indexing
                      n636 = Enqueue Element(queue=w1851, element=w1849) -> (queue out=w1850:refnum<queue>)  [unwired: 2 in, 2 out]
                    }
                  }
                }
                n637 = Or(x=w1834, y=w1833) -> (x .or. y?=w1836:bool)
                n638 = Select(t=State_Type_Definitions,_for_0.26g_versions_and_later_2."True Stop" ("Enum"), s=w1833, f=State_Type_Definitions,_for_0.26g_versions_and_later_2."Task 8J: CLOSE CLAW" ("Enum")) -> (s? t:f=w1830:T18)
                n639 = Select(t=w1830, s=w1836, f=State_Type_Definitions,_for_0.26g_versions_and_later_2."Task 8I: ARM GRAB HEIGHT" ("Enum")) -> (s? t:f=w1835:T18)
              }
              frame "Exit" {
                n640 = for {
                  shift-right: [w1858] -> w1855
                  shift-left: w1852 -> [w1859]
                  tunnel: string[] ["STOP", "RESET ENCODERS", "RESET YAW", "ARDUINO MODE 0"] -> [w1857] mode=indexing
                  n641 = Enqueue Element(queue=w1859, element=w1857) -> (queue out=w1858:refnum<queue>)  [unwired: 2 in, 2 out]
                }
              }
            }
          }
          frame 36 {
            # ">>> yStepper command>>>"
            # ">> Manual override >>"
            n642 = Dequeue Element(queue=w1870, timeout in ms (-1)=w1869, error in (no error)=w1868) -> (element=w1867:T10)  [unwired: 3 out]
            n643 = case shown="\"Start Task 1\", Default" w1867 {
              tunnel: [w1879 State_Type_Definitions,_for_0.26g_versions_and_later_2."True Stop" ("Enum")] -> w1872
              tunnel: [w1882 w1899] -> w1865
              tunnel: [State_Type_Definitions,_for_0.26g_versions_and_later_2."Idle" ("Enum") State_Type_Definitions,_for_0.26g_versions_and_later_2."Shutdown" ("Enum")] -> w1864
              tunnel: w1866 -> [w1873 _]
              tunnel: w1871 -> [w1878 w1896]
              tunnel: w1862 -> [w1877 _]
              frame "Start Task 1", Default {
                # ">> Is time up? >>"
                # "Determines if object is in range to pick up"
                # ">> Manual override >>"
                n644 = case shown="True" w1877 {
                  tunnel: [w1886 w1892] -> w1882